vi "HFRR ADV v037.vi"() -> ()   [LabVIEW 2025] (continued)
                w348 = "" ("FILE")
                n261 = local write "Main Tab"(T2."Adv Scar" ("Main Tab")) -> ()
                n262 = local write "measured_stroke"(0.0 ("measured_stroke")) -> ()
                n263 = local write "Main Dashboard Buttons"(T1."Imaging" ("Main Dashboard Buttons")) -> ()
                n264 = property on="RUN" class="Bool (strict)"("Visible"=TRUE) -> ()  [unwired: 2 in, 2 out]
                n265 = local write "Due Write"("VC;0") -> ()
                n266 = local write "Humidity"(TRUE ("Humidity")) -> ()
                n267 = local write "TEST FILE NAM,E SAVED"(FALSE ("TEST FILE NAM,E SAVED")) -> ()
                n268 = local write "Fuel Discription :"(w348) -> ()
                n269 = local write "Batch Ref Num :"(w348) -> ()
                n270 = local write "Remarks :"(w348) -> ()
                n271 = local write "FILE"(w348) -> ()
                n272 = property on="FRICVALZ 2" class="Bool (strict)"("DisabledEnum"=w347) -> ()  [unwired: 2 in, 2 out]
                n273 = property on="FRICVALZ 4" class="Bool (strict)"("DisabledEnum"=w347) -> ()  [unwired: 2 in, 2 out]
                n274 = property on="FRICVALZ 3" class="Bool (strict)"("DisabledEnum"=w347) -> ()  [unwired: 2 in, 2 out]
              }
            }
          }
          frame True {
            n275 = stacked-sequence {
              frame #0 {
                n276 = local write "Due Write"("DAC;200") -> ()
              }
              frame #1 {
                n277 = Wait (ms)(milliseconds to wait=u32 1500) -> ()  [unwired: 1 out]
              }
              frame #2 {
                n278 = local write "Due Write"("DAC;200") -> ()
              }
              frame #3 {
                n279 = Wait (ms)(milliseconds to wait=u32 1000) -> ()  [unwired: 1 out]
              }
              frame #4 {
                n280 = local write "Due Write"("VC;1") -> ()
              }
              frame #5 {
                n281 = Wait (ms)(milliseconds to wait=u32 2000) -> ()  [unwired: 1 out]
              }
              frame #6 {
                n282 = local write "Due Write"("VC;1") -> ()
              }
              frame #7 {
                n283 = Wait (ms)(milliseconds to wait=u32 2000) -> ()  [unwired: 1 out]
              }
              frame #8 {
                w359 = T19."Disabled" ("Disabled")
                n284 = property on="RUN" class="Bool (strict)"("Visible"=FALSE) -> ()  [unwired: 2 in, 2 out]
                n285 = property on="FRICVALZ 2" class="Bool (strict)"("DisabledEnum"=w359) -> ()  [unwired: 2 in, 2 out]
                n286 = property on="FRICVALZ 4" class="Bool (strict)"("DisabledEnum"=w359) -> ()  [unwired: 2 in, 2 out]
                n287 = property on="FRICVALZ 3" class="Bool (strict)"("DisabledEnum"=w359) -> ()  [unwired: 2 in, 2 out]
                "START TEMP" <- TRUE
              }
            }
          }
        }
      }
      event "FILE", "USERNAME", "USER ID": Mouse Enter {
        n288 = event-data() -> ()  [unwired: 1 in, 4 out]
        n289 = dll-call lib="kernel32.dll" fn="Wow64DisableWow64FsRedirection"("OldValue"=0) -> (error out=w366:errorcluster, "OldValue"=w364:i32)  [unwired: 4 in, 1 out]
        n290 = call <vilib>:"System Exec.vi"("run minimized? (F)"=TRUE, "error in (no error)"=w366, "command line"="C:\\Program Files\\Common Files\\Microsoft Shared\\Ink\\TabTip.exe") -> ("error out"=w365:errorcluster)  [unwired: 5 in, 3 out]
        n291 = dll-call lib="kernel32.dll" fn="Wow64EnableWow64FsRedirection"(error in=w365, "OldValue"=w364) -> ()  [unwired: 4 in, 2 out]
      }
      event "EDIT": Value Change {
        n292 = event-data() -> ()  [unwired: 1 in, 6 out]
        n293 = local read "EDIT"() -> (w367:bool)
        n294 = case shown="False" w367 {
          frame False {
            n295 = control-ref of="This VI"() -> (w384:refnum<vi>)
            n296 = property class="VI"(reference=w384) -> (reference out=w375:refnum<vi>, error out=w379:errorcluster, "Panel"=w383:refnum<vi>)  [unwired: 1 in]
            n297 = property class="Pnl"(reference=w383, error in=w379) -> (reference out=w377:refnum<vi>, error out=w380:errorcluster, "Panes[]"=w382:refnum<vi>[])
            n298 = for {
              tunnel: w382 -> [w390] mode=indexing
              tunnel: T24."Always Off" ("Horizontal Scrollbar Visibility") -> [w389]
              tunnel: w380 -> [w386]
              tunnel: [w385] -> w378
              n299 = property class="Pane"(reference=w390, error in=w386, "HorizScrollbarVisibility"=w389) -> (reference out=w387:refnum<vi>, error out=w388:errorcluster)
              n300 = Close Reference(reference=w387, error in (no error)=w388) -> (error out=w385:errorcluster)
            }
            n301 = Close Reference(reference=w377, error in (no error)=w378) -> (error out=w376:errorcluster)
            n302 = Close Reference(reference=w375, error in (no error)=w376) -> (error out=w370:errorcluster)
            "error out 7" <- w370
            n303 = call <vilib>:"Clear Errors.vi"("error in (no error)"=w370) -> ("error out"=w369:errorcluster)  [unwired: 5 in, 1 out]
            n304 = local write "Service Password enable"(FALSE ("Service Password enable")) -> ()
            n305 = call <userlib>:"Fit VI window to Largest Dec.vi"("error in (no error)"=w369, "border spacing (2 px)"=1) -> ("error out"=w374:errorcluster, "dup VI Ref"=w372:refnum<vi>)  [unwired: 4 in]
            n306 = invoke on="Invoke Node" class="VI" method="FP.Run-Time Position.Maximized"(reference=w372, error in=w374) -> (error out=w373:errorcluster)  [unwired: 2 in, 3 out]
            n307 = call <vilib>:"Clear Errors.vi"("error in (no error)"=w373) -> ()  [unwired: 5 in, 2 out]
          }
          frame True {
          }
        }
      }
      event "Heater Button": Value Change {
        n308 = event-data() -> ()  [unwired: 1 in, 6 out]
        n309 = local read "Heater Button"() -> (w391:bool)
        n310 = case shown="True" w391 {
          frame True {
            n311 = stacked-sequence {
              frame #0 {
                n312 = Wait (ms)(milliseconds to wait=u32 1500) -> ()  [unwired: 1 out]
              }
              frame #1 {
                n313 = local read "Set Temp"() -> (w393:dbl)
                n314 = Number To Fractional String(number=w393, precision (6)=i16 2) -> (F-format string=w396:string)  [unwired: 2 in]
                n315 = Concatenate Strings("ST;" ("Command"), w396) -> (w395:string)
                n316 = local write "Due Write"(w395) -> ()
              }
              frame #2 {
                n317 = Wait (ms)(milliseconds to wait=u32 1500) -> ()  [unwired: 1 out]
              }
              frame #3 {
                n318 = local write "Due Write"("HE;1" ("Command")) -> ()
              }
              frame #4 {
                n319 = Wait (ms)(milliseconds to wait=u32 1500) -> ()  [unwired: 1 out]
              }
              frame #5 {
                n320 = stacked-sequence {
                  frame #0 {
                    n321 = Wait (ms)(milliseconds to wait=u32 1500) -> ()  [unwired: 1 out]
                  }
                  frame #1 {
                    n322 = local read "Set Temp"() -> (w402:dbl)
                    n323 = Number To Fractional String(number=w402, precision (6)=i16 2) -> (F-format string=w405:string)  [unwired: 2 in]
                    n324 = Concatenate Strings("ST;" ("Command"), w405) -> (w404:string)
                    n325 = local write "Due Write"(w404) -> ()
                  }
                  frame #2 {
                    n326 = Wait (ms)(milliseconds to wait=u32 1500) -> ()  [unwired: 1 out]
                  }
                  frame #3 {
                    n327 = local write "Due Write"("HE;1" ("Command")) -> ()
                  }
                  frame #4 {
                    n328 = Wait (ms)(milliseconds to wait=u32 1500) -> ()  [unwired: 1 out]
                  }
                }
              }
            }
          }
          frame False {
            n329 = stacked-sequence {
              frame #0 {
                n330 = Wait (ms)(milliseconds to wait=u32 1500) -> ()  [unwired: 1 out]
              }
              frame #1 {
                n331 = Concatenate Strings("ST;" ("Command"), "0" ("string")) -> (w412:string)
                n332 = local write "Due Write"(w412) -> ()
              }
              frame #2 {
                n333 = Wait (ms)(milliseconds to wait=u32 1500) -> ()  [unwired: 1 out]
              }
              frame #3 {
                n334 = local write "Due Write"("HE;0" ("Command")) -> ()
              }
              frame #4 {
                n335 = Wait (ms)(milliseconds to wait=u32 1500) -> ()  [unwired: 1 out]
              }
            }
          }
        }
      }
      event "Headen Service Button": Value Change {
        n336 = event-data() -> ()  [unwired: 1 in, 6 out]
        n337 = local read "Headen Service Button"() -> (w417:bool)
        n338 = case shown="True" w417 {
          frame False {
            n339 = property on="Password 3" class="Clust (strict)"("Visible"=FALSE) -> ()  [unwired: 2 in, 2 out]
            n340 = property on="Service Password Log" class="Str"("Visible"=FALSE) -> ()  [unwired: 2 in, 2 out]
          }
          frame True {
            n341 = property on="Password 3" class="Clust (strict)"("Visible"=TRUE) -> ()  [unwired: 2 in, 2 out]
            n342 = property on="Service Password Log" class="Str"("Visible"=TRUE) -> ()  [unwired: 2 in, 2 out]
          }
        }
      }
      event "Password 3.Service Password": Value Change {
        n343 = event-data() -> ()  [unwired: 1 in, 6 out]
        n344 = Unbundle By Name("Password 3") -> ("Service Password"=w424:string)
        n345 = call <vilib>:"Trim Whitespace.vi"("string"=w424) -> ("trimmed string"=w422:string)  [unwired: 1 in]
        n346 = Equal?(x=w422, y="Service@123") -> (x = y?=w423:bool)
        n347 = case shown="False" w423 {
          selector: w423 -> [w427 w429]
          frame False {
            n348 = local write "Service Password enable"(w427) -> ()
            n349 = property on="Service Password Log" class="Str"("Visible"=TRUE) -> ()  [unwired: 2 in, 2 out]
          }
          frame True {
            n350 = property on="Service Password Log" class="Str"("Visible"=FALSE) -> ()  [unwired: 2 in, 2 out]
            "Service Password enable" <- w429
          }
        }
      }
      event "Sign In": Value Change {
        w431 = FALSE ("Visible")
        n351 = event-data() -> ()  [unwired: 1 in, 6 out]
        n352 = property on="About" class="Clust (strict)"("Visible"=w431) -> ()  [unwired: 2 in, 2 out]
        n353 = property on="Password 3" class="Clust (strict)"("Visible"=w431) -> ()  [unwired: 2 in, 2 out]
        n354 = property on="Service Password Log" class="Str"("Visible"=FALSE) -> ()  [unwired: 2 in, 2 out]
      }
      event "Info": Value Change {
        n355 = event-data() -> ()  [unwired: 1 in, 6 out]
        n356 = local read "Info"() -> (w433:bool)
        n357 = case shown="False" w433 {
          frame False {
            n358 = property on="About" class="Clust (strict)"("Visible"=FALSE) -> ()  [unwired: 2 in, 2 out]
          }
          frame True {
            n359 = property on="About" class="Clust (strict)"("Visible"=TRUE) -> ()  [unwired: 2 in, 2 out]
          }
        }
      }
      event "Calibration": Value Change {
        n360 = event-data() -> ()  [unwired: 1 in, 6 out]
        n361 = local read "Calibration"() -> (w437:bool)
        n362 = case shown="False" w437 {
          frame False {
            n363 = property on="Calibration 2" class="TabCtl (strict)"("Visible"=FALSE) -> ()  [unwired: 2 in, 2 out]
            n364 = local write "Cal Password"("" ("Cal Password")) -> ()
          }
          frame True {
            n365 = property on="Calibration 2" class="TabCtl (strict)"("Visible"=TRUE) -> ()  [unwired: 2 in, 2 out]
            n366 = local write "Cal Password"("" ("Cal Password")) -> ()
          }
        }
        n367 = property on="Wrong Password" class="Str"("Visible"=FALSE) -> ()  [unwired: 2 in, 2 out]
      }
      event "Cal Password": Value Change {
        n368 = event-data() -> ()  [unwired: 1 in, 6 out]
        n369 = local read "Cal Password"() -> (w445:string)
        n370 = call <vilib>:"Trim Whitespace.vi"("string"=w445) -> ("trimmed string"=w444:string)  [unwired: 1 in]
        n371 = Equal?(x=w444, y="Cal@321") -> (x = y?=w442:bool)
        n372 = case shown="True" w442 {
          frame False {
            n373 = property on="Wrong Password" class="Str"("Visible"=TRUE) -> ()  [unwired: 2 in, 2 out]
          }
          frame True {
            n374 = property on="Wrong Password" class="Str"("Visible"=FALSE) -> ()  [unwired: 2 in, 2 out]
            n375 = local write "Main Tab"(T2."About" ("Main Tab")) -> ()
            n376 = local write "Cal Password"("" ("Cal Password")) -> ()
            n377 = local write "Main Dashboard Buttons"(T1."About" ("Main Dashboard Buttons")) -> ()
            n378 = property on="Calibration 2" class="TabCtl (strict)"("Visible"=FALSE) -> ()  [unwired: 2 in, 2 out]
            n379 = local write "Calibration"(FALSE ("Calibration")) -> ()
          }
        }
      }
      event "Calibration Selection": Value Change {
        n380 = event-data() -> ()  [unwired: 1 in, 6 out]
        n381 = local read "Calibration Selection"() -> (w454:T8)
        n382 = case shown="\"Stroke Calibration\"" w454 {
          tunnel: [T7."Stroke" ("Main Calibration Tab") T7."Friction" ("Main Calibration Tab") T7."Main" ("Main Calibration Tab") T7."Temperature" ("Main Calibration Tab")] -> w453
          frame "Stroke Calibration" {
          }
          frame "Friction Force Calibration" {
          }
          frame Default {
          }
          frame "Temperature Calibration" {
          }
        }
        n383 = local write "Main Calibration Tab"(w453) -> ()
      }
      event "Back Stroke": Value Change {
        n384 = event-data() -> ()  [unwired: 1 in, 6 out]
        n385 = local write "Main Stroke Tab"(T9."Step 1" ("Main Stroke Tab")) -> ()
        n386 = local write "Main Calibration Tab"(T7."Main" ("Main Calibration Tab")) -> ()
        n387 = local write "Back Stroke"(FALSE ("Back Stroke")) -> ()
      }
      event "Step 2 Back": Value Change {
        n388 = event-data() -> ()  [unwired: 1 in, 6 out]
        n389 = local write "Main Stroke Tab"(T9."Step 1" ("Main Stroke Tab")) -> ()
        n390 = local write "Step 2 Back"(FALSE ("Back Stroke")) -> ()
      }
      event "Step 3 Back": Value Change {
        n391 = event-data() -> ()  [unwired: 1 in, 6 out]
        n392 = local write "Main Stroke Tab"(T9."Step 2" ("Main Stroke Tab")) -> ()
        n393 = local write "Step 3 Back"(FALSE ("Back Stroke")) -> ()
      }
      event "Step 4 Back": Value Change {
        n394 = event-data() -> ()  [unwired: 1 in, 6 out]
        n395 = local write "Main Stroke Tab"(T9."Step 3" ("Main Stroke Tab")) -> ()
        n396 = local write "Step 4 Back"(FALSE ("Back Stroke")) -> ()
      }
      event "Step 5 Back": Value Change {
        n397 = event-data() -> ()  [unwired: 1 in, 6 out]
        n398 = local write "Main Stroke Tab"(T9."Step 4" ("Main Stroke Tab")) -> ()
        n399 = local write "Step 5 Back"(FALSE ("Back Stroke")) -> ()
      }
      event "Step 6 Back": Value Change {
        n400 = event-data() -> ()  [unwired: 1 in, 6 out]
        n401 = local write "Main Stroke Tab"(T9."Step 5" ("Main Stroke Tab")) -> ()
        n402 = local write "Step 6 Back"(FALSE ("Back Stroke")) -> ()
      }
      event "Back Stroke step 7": Value Change {
        n403 = event-data() -> ()  [unwired: 1 in, 6 out]
        n404 = local write "Main Stroke Tab"(T9."Step 6" ("Main Stroke Tab")) -> ()
        n405 = local write "Back Stroke step 7"(FALSE ("Back Stroke")) -> ()
      }
      event "Back Stroke step 8": Value Change {
        n406 = event-data() -> ()  [unwired: 1 in, 6 out]
        n407 = local write "Main Stroke Tab"(T9."Step 7" ("Main Stroke Tab")) -> ()
        n408 = local write "Back Stroke step 8"(FALSE ("Back Stroke")) -> ()
      }
      event "Back Stroke 8": Value Change {
        n409 = event-data() -> ()  [unwired: 1 in, 6 out]
        n410 = local write "MOVE CARRIAGE TO"(0.2 ("MOVE CARRIAGE TO")) -> ()
        n411 = local write "Main Stroke Tab"(T9."Step 1" ("Main Stroke Tab")) -> ()
        n412 = local write "Back Stroke 8"(FALSE ("Back Stroke 8")) -> ()
      }
      event "Continue Stroke": Value Change {
        n413 = event-data() -> ()  [unwired: 1 in, 6 out]
        n414 = local write "Main Stroke Tab"(T9."Step 2" ("Main Stroke Tab")) -> ()
        n415 = local write "Continue Stroke"(FALSE ("Continue Stroke")) -> ()
      }
      event "Continue Stroke step 2": Value Change {
        n416 = event-data() -> ()  [unwired: 1 in, 6 out]
        n417 = local write "Main Stroke Tab"(T9."Step 3" ("Main Stroke Tab")) -> ()
        n418 = local write "Continue Stroke step 2"(FALSE ("Continue Stroke")) -> ()
      }
      event "Continue Stroke step 3": Value Change {
        n419 = event-data() -> ()  [unwired: 1 in, 6 out]
        n420 = local write "Main Stroke Tab"(T9."Step 4" ("Main Stroke Tab")) -> ()
        n421 = local write "Continue Stroke step 3"(FALSE ("Continue Stroke")) -> ()
      }
      event "Continue Stroke step 4": Value Change {
        n422 = event-data() -> ()  [unwired: 1 in, 6 out]
        n423 = local write "Main Stroke Tab"(T9."Step 5" ("Main Stroke Tab")) -> ()
        n424 = local write "Continue Stroke step 4"(FALSE ("Continue Stroke")) -> ()
      }
      event "Continue Stroke step 5": Value Change {
        n425 = event-data() -> ()  [unwired: 1 in, 6 out]
        n426 = local write "Main Stroke Tab"(T9."Step 6" ("Main Stroke Tab")) -> ()
        n427 = local write "Continue Stroke step 5"(FALSE ("Continue Stroke")) -> ()
      }
      event "Continue Stroke step 6": Value Change {
        n428 = event-data() -> ()  [unwired: 1 in, 6 out]
        n429 = local write "Main Stroke Tab"(T9."Step 7" ("Main Stroke Tab")) -> ()
        n430 = local write "Continue Stroke step 6"(FALSE ("Continue Stroke")) -> ()
      }
      event "Continue Stroke step 7": Value Change {
        w493 = FALSE ("0.2mm")
        n431 = event-data() -> ()  [unwired: 1 in, 6 out]
        n432 = local write "0.4 mm"(w493) -> ()
        n433 = local write "0.6 mm"(w493) -> ()
        n434 = local write "1.0 mm"(w493) -> ()
        n435 = local write "1.2 mm"(w493) -> ()
        n436 = local write "0.2 2"(w493) -> ()
        n437 = local write "0.4 2"(w493) -> ()
        n438 = local write "0.6 2"(w493) -> ()
        n439 = local write "0.8 2"(w493) -> ()
        n440 = local write "1.0 2"(w493) -> ()
        n441 = local write "1.2"(w493) -> ()
        n442 = local write "0.2mm"(w493) -> ()
        n443 = local write "0.8mm"(w493) -> ()
        n444 = local write "Main Stroke Tab"(T9."Step 8" ("Main Stroke Tab")) -> ()
        n445 = local write "Continue Stroke step 7"(FALSE ("Continue Stroke")) -> ()
        n446 = local write "Stroke Test Complete"(T10."Test Progress" ("Stroke Test Complete")) -> ()
        "Position Measurment Temp" <- 0.0 ("Position Measurment Temp")
        "Calibration Tare" <- TRUE ("Calibration Tare")
        "MOVE CARRIAGE TO" <- 0.2 ("MOVE CARRIAGE TO")
      }
      event "Continue Stroke step 8": Value Change {
        n447 = event-data() -> ()  [unwired: 1 in, 6 out]
        n448 = local read "LVDT STROKE  Calibration"() -> (w498:dbl)
        n449 = local read "Position Measurment Temp"() -> (w499:dbl)
        n450 = case shown="7" w499 {
          selector: w499 -> [w504 w509 w514 w519 w524 w528 w531 w532]
          tunnel: w498 -> [w500 w505 w510 w515 w520 w525 _ _]
          frame 0, Default {
            w502 = TRUE ("0.2mm")
            n451 = Increment(x=w504) -> (x+1=w503:i32)
            n452 = local write "Position Measurment Temp"(w503) -> ()
            n453 = local write "0.2mm"(w502) -> ()
            n454 = local write "0.2 2"(w502) -> ()
            n455 = local write "MOVE CARRIAGE TO"(0.4 ("MOVE CARRIAGE TO")) -> ()
            "Calibration 0.2" <- w500
          }
          frame 1 {
            w507 = TRUE ("0.4 mm")
            n456 = Increment(x=w509) -> (x+1=w508:i32)
            n457 = local write "Calibration 0.4"(w505) -> ()
            n458 = local write "Position Measurment Temp"(w508) -> ()
            n459 = local write "0.4 mm"(w507) -> ()
            n460 = local write "MOVE CARRIAGE TO"(0.6 ("MOVE CARRIAGE TO")) -> ()
            n461 = local write "0.4 2"(w507) -> ()
          }
          frame 2 {
            w512 = TRUE ("0.6 mm")
            n462 = Increment(x=w514) -> (x+1=w513:i32)
            n463 = local write "Calibration 0.6"(w510) -> ()
            n464 = local write "Position Measurment Temp"(w513) -> ()
            n465 = local write "0.6 2"(w512) -> ()
            n466 = local write "0.6 mm"(w512) -> ()
            n467 = local write "MOVE CARRIAGE TO"(0.8 ("MOVE CARRIAGE TO")) -> ()
          }
          frame 3 {
            w516 = TRUE ("0.6 mm")
            n468 = Increment(x=w519) -> (x+1=w518:i32)
            n469 = local write "Position Measurment Temp"(w518) -> ()
            n470 = local write "MOVE CARRIAGE TO"(1.0 ("MOVE CARRIAGE TO")) -> ()
            n471 = local write "0.8mm"(w516) -> ()
            n472 = local write "0.8 2"(w516) -> ()
            "Calibration 0.8" <- w515
          }
          frame 4 {
            w521 = TRUE ("0.6 mm")
            n473 = Increment(x=w524) -> (x+1=w523:i32)
            n474 = local write "Position Measurment Temp"(w523) -> ()
            n475 = local write "MOVE CARRIAGE TO"(1.2 ("MOVE CARRIAGE TO")) -> ()
            n476 = local write "1.0 mm"(w521) -> ()
            n477 = local write "1.0 2"(w521) -> ()
            "Calibration 1.0" <- w520
          }
          frame 5 {
            w526 = TRUE ("0.6 mm")
            n478 = Increment(x=w528) -> (x+1=w527:i32)
            n479 = local write "Position Measurment Temp"(w527) -> ()
            n480 = local write "1.2 mm"(w526) -> ()
            n481 = local write "1.2"(w526) -> ()
            "Calibration 1.2" <- w525
          }
          frame 6 {
            n482 = Increment(x=w531) -> (x+1=w530:i32)
            n483 = local write "Position Measurment Temp"(w530) -> ()
            n484 = local write "Stroke Test Complete"(T10."Stroke Points Completed" ("Stroke Test Complete")) -> ()
          }
          frame 7 {
            n485 = stacked-sequence {
              tunnel: w532 -> [w533 _ _]
              frame #0 {
                n486 = Increment(x=w533) -> (x+1=w534:i32)
                n487 = local write "Main Stroke Tab"(T9."Step 9" ("Main Stroke Tab")) -> ()
                n488 = local write "Position Measurment Temp"(w534) -> ()
                n489 = Insert Into Array(array=dbl[] [], new element #1=0.2 ("new element/subarray"), new element #2=0.4 ("new element/subarray"), new element #3=0.6 ("new element/subarray"), new element #4=0.8 ("new element/subarray"), new element #5=1.0 ("new element/subarray"), new element #6=1.2 ("new element/subarray")) -> (→"1D stroke":dbl[])  [unwired: 1 in]
                n490 = local read "Calibration 0.2"() -> (w541:dbl)
                n491 = local read "Calibration 0.4"() -> (w540:dbl)
                n492 = local read "Calibration 0.6"() -> (w539:dbl)
                n493 = local read "Calibration 0.8"() -> (w538:dbl)
                n494 = local read "Calibration 1.0"() -> (w537:dbl)
                n495 = local read "Calibration 1.2"() -> (w536:dbl)
                n496 = Insert Into Array(array=dbl[] [], new element #1=w541, new element #2=w540, new element #3=w539, new element #4=w538, new element #5=w537, new element #6=w536) -> (→"Calibrated Voltage Value":dbl[])  [unwired: 1 in]
              }
              frame #1 {
                n497 = local read "calibration values"() -> (w564:dbl[])
                n498 = local read "Calibrated Voltage Value"() -> (w566:dbl[])
                n499 = Index Array(array=w564, index #1=1 ("index"), index #2=3 ("index"), index #3=5 ("index"), index #4=7 ("index"), index #5=9 ("index"), index #6=11 ("index")) -> (element #1=w557:dbl, element #2=w556:dbl, element #3=w555:dbl, element #4=w554:dbl, element #5=w553:dbl, element #6=w552:dbl)
                n500 = local read "1D stroke"() -> (w567:dbl[])
                n501 = for {
                  tunnel: [w576] -> w565 mode=indexing
                  tunnel: w567 -> [w575] mode=indexing
                  tunnel: w566 -> [w574] mode=indexing
                  tunnel: w557 -> [w573]
                  tunnel: w556 -> [w572]
                  tunnel: w555 -> [w571]
                  tunnel: w554 -> [w570]
                  tunnel: w553 -> [w569]
                  tunnel: w552 -> [w568]
                  n502 = formula code="if (stroke == 0.2)\n{\n    if ((voltage >= REF_02 - 0.2) && (voltage <= REF_02 + 0.2))\n        status = 1;\n    else\n        status = 0;\n}\nelse if (stroke == 0.4)\n{\n    if ((voltage >= REF_04 - 0.2) && (voltage <= REF_04 + 0.2))\n        status = 1;\n    else\n        status = 0;\n}\nelse if (stroke == 0.6)\n{\n    if ((voltage >= REF_06 - 0.2) && (voltage <= REF_06 + 0.2))\n        status = 1;\n    else\n        status = 0;\n}\nelse if (stroke == 0.8)\n{\n    if ((voltage >= REF_08 - 0.2) && (voltage <= REF_08 + 0.2))\n        status = 1;\n    else\n        status = 0;\n}\nelse if (stroke == 1.0)\n{\n    if ((voltage >= REF_10 - 0.2) && (voltage <= REF_10 + 0.2))\n        status = 1;\n    else\n        status = 0;\n}\nelse if (stroke == 1.2)\n{\n    if ((voltage >= REF_12 - 0.2) && (voltage <= REF_12 + 0.2))\n        status = 1;\n    else\n        status = 0;\n}\nelse\n{\n    status = 0;\n}"("stroke"=w575, "voltage"=w574, "REF_02"=w573, "REF_04"=w572, "REF_06"=w571, "REF_08"=w570, "REF_10"=w569, "REF_12"=w568) -> ("status"=w576:dbl)
                }
                "Status" <- w565
              }
              frame #2 {
                w583 = 1.0
                n503 = local read "Status"() -> (w590:dbl[])
                n504 = Index Array(array=w590) -> (element #1=w589:dbl, element #2=w588:dbl, element #3=w587:dbl, element #4=w586:dbl, element #5=w585:dbl, element #6=w584:dbl)  [unwired: 6 in]
                n505 = Equal?(x=w588, y=w583) -> (x = y?=w581:bool)
                n506 = Equal?(x=w587, y=w583) -> (x = y?=w580:bool)
                n507 = Equal?(x=w586, y=w583) -> (x = y?=w579:bool)
                n508 = Equal?(x=w585, y=w583) -> (x = y?=w578:bool)
                n509 = Equal?(x=w584, y=w583) -> (x = y?=w577:bool)
                n510 = Equal?(x=w589, y=w583) -> (x = y?=w582:bool)
                n511 = case shown="True" w582 {
                  selector: w582 -> [w601 w602]
                  frame True {
                    n512 = local write "Point 1 - 0.2 mm"(w601) -> ()
                    n513 = property on="Point 1 - 0.2 mm" class="Bool"("Caption.Visible"=w601) -> ()  [unwired: 2 in, 2 out]
                  }
                  frame False {
                    n514 = local write "Point 1 - 0.2 mm"(w602) -> ()
                    n515 = property on="Point 1 - 0.2 mm" class="Bool"("Caption.Visible"=w602) -> ()  [unwired: 2 in, 2 out]
                  }
                }
                n516 = case shown="True" w581 {
                  selector: w581 -> [w599 w600]
                  frame True {
                    n517 = local write "Point 2 - 0.4 mm"(w599) -> ()
                    n518 = property on="Point 2 - 0.4 mm" class="Bool"("Caption.Visible"=w599) -> ()  [unwired: 2 in, 2 out]
                  }
                  frame False {
                    n519 = local write "Point 2 - 0.4 mm"(w600) -> ()
                    n520 = property on="Point 2 - 0.4 mm" class="Bool"("Caption.Visible"=w600) -> ()  [unwired: 2 in, 2 out]
                  }
                }
                n521 = case shown="True" w578 {
                  selector: w578 -> [w593 w594]
                  frame True {
                    n522 = local write "Point 5 - 1.0 mm"(w593) -> ()
                    n523 = property on="Point 5 - 1.0 mm" class="Bool"("Caption.Visible"=w593) -> ()  [unwired: 2 in, 2 out]
                  }
                  frame False {
                    n524 = local write "Point 5 - 1.0 mm"(w594) -> ()
                    n525 = property on="Point 5 - 1.0 mm" class="Bool"("Caption.Visible"=w594) -> ()  [unwired: 2 in, 2 out]
                  }
                }
                n526 = case shown="True" w580 {
                  selector: w580 -> [w597 w598]
                  frame True {
                    n527 = local write "Point 3 - 0.6 mm"(w597) -> ()
                    n528 = property on="Point 3 - 0.6 mm" class="Bool"("Caption.Visible"=w597) -> ()  [unwired: 2 in, 2 out]
                  }
                  frame False {
                    n529 = local write "Point 3 - 0.6 mm"(w598) -> ()
                    n530 = property on="Point 3 - 0.6 mm" class="Bool"("Caption.Visible"=w598) -> ()  [unwired: 2 in, 2 out]
                  }
                }
                n531 = case shown="True" w579 {
                  selector: w579 -> [w595 w596]
                  frame True {
                    n532 = local write "Point 4 - 0.8 mm"(w595) -> ()
                    n533 = property on="Point 4 - 0.8 mm" class="Bool"("Caption.Visible"=w595) -> ()  [unwired: 2 in, 2 out]
                  }
                  frame False {
                    n534 = local write "Point 4 - 0.8 mm"(w596) -> ()
                    n535 = property on="Point 4 - 0.8 mm" class="Bool"("Caption.Visible"=w596) -> ()  [unwired: 2 in, 2 out]
                  }
                }
                n536 = case shown="True" w577 {
                  selector: w577 -> [w591 w592]
                  frame True {
                    n537 = local write "Point 6 - 1.2 mm"(w591) -> ()
                    n538 = property on="Point 6 - 1.2 mm" class="Bool"("Caption.Visible"=w591) -> ()  [unwired: 2 in, 2 out]
                  }
                  frame False {
                    n539 = local write "Point 6 - 1.2 mm"(w592) -> ()
                    n540 = property on="Point 6 - 1.2 mm" class="Bool"("Caption.Visible"=w592) -> ()  [unwired: 2 in, 2 out]
                  }
                }
              }
            }
          }
        }
      }
      event "TEMPERATURE STEP Back 1", "TEMPERATURE STEP Back air Temp": Value Change {
        n541 = event-data() -> ()  [unwired: 1 in, 6 out]
        n542 = stacked-sequence {
          frame #0 {
            n543 = local write "Main Calibration Tab"(T7."Main" ("Main Calibration Tab")) -> ()
          }
          frame #1 {
            n544 = Wait (ms)(milliseconds to wait=u32 1000) -> ()  [unwired: 1 out]
          }
          frame #2 {
            n545 = local write "Due Write"("CAL;END" ("Command")) -> ()
          }
          frame #3 {
            n546 = Wait (ms)(milliseconds to wait=u32 2000) -> ()  [unwired: 1 out]
          }
          frame #4 {
            n547 = local write "Due Write"("CAL;END" ("Command")) -> ()
          }
        }
      }
      event "Temperature Continue Step 1": Value Change {
        n548 = event-data() -> ()  [unwired: 1 in, 6 out]
        n549 = stacked-sequence {
          frame #0 {
            n550 = Wait (ms)(milliseconds to wait=u32 1500) -> ()  [unwired: 1 out]
          }
          frame #1 {
            n551 = local write "Due Write"("CAL;START" ("Command")) -> ()
          }
          frame #2 {
            n552 = Wait (ms)(milliseconds to wait=u32 1500) -> ()  [unwired: 1 out]
          }
          frame #3 {
            n553 = local write "Due Write"("CAL;START" ("Command")) -> ()
          }
          frame #4 {
            n554 = Wait (ms)(milliseconds to wait=u32 2000) -> ()  [unwired: 1 out]
          }
          frame #5 {
          }
          frame #6 {
            n555 = Wait (ms)(milliseconds to wait=u32 2000) -> ()  [unwired: 1 out]
          }
          frame #7 {
            # "CAL;A1;<true_T>"
            n556 = local write "Due Write"("CAL;A1;0" ("Command")) -> ()
          }
          frame #8 {
            n557 = local write "Tab Control 4"(T12."Step 2" ("Tab Control 4")) -> ()
          }
        }
      }
      event "Temperature Continue Step air Step 1": Value Change {
        n558 = event-data() -> ()  [unwired: 1 in, 6 out]
        n559 = stacked-sequence {
          frame #0 {
            n560 = Wait (ms)(milliseconds to wait=u32 1500) -> ()  [unwired: 1 out]
          }
          frame #1 {
            n561 = local write "Due Write"("CAL;START" ("Command")) -> ()
          }
          frame #2 {
            n562 = Wait (ms)(milliseconds to wait=u32 1500) -> ()  [unwired: 1 out]
          }
          frame #3 {
            n563 = local write "Due Write"("CAL;START" ("Command")) -> ()
          }
          frame #4 {
            n564 = Wait (ms)(milliseconds to wait=u32 2000) -> ()  [unwired: 1 out]
          }
          frame #5 {
          }
          frame #6 {
            n565 = Wait (ms)(milliseconds to wait=u32 2000) -> ()  [unwired: 1 out]
          }
          frame #7 {
            # "CAL;A1;<true_T>"
            n566 = local write "Due Write"("CAL;A1;0" ("Command")) -> ()
          }
          frame #8 {
            n567 = local write "Tab Control 4"(T12."Air Step 2" ("Tab Control 4")) -> ()
          }
        }
      }
      event "Temperature Selection": Value Change {
        n568 = event-data() -> ()  [unwired: 1 in, 6 out]
        n569 = local read "Temperature Selection"() -> (w624:T13)
        n570 = case shown="\"Sample Temperature\"" w624 {
          frame "Air Temperature" {
            n571 = local write "Tab Control 4"(T12."Air Step 1" ("Tab Control 4")) -> ()
          }
          frame "Sample Temperature" {
            n572 = local write "Tab Control 4"(T12."Step 1" ("Tab Control 4")) -> ()
          }
          frame "Default", Default {
          }
        }
      }
      event "Temperature Continue Step 2": Value Change {
        n573 = event-data() -> ()  [unwired: 1 in, 6 out]
        n574 = stacked-sequence {
          frame #0 {
            n575 = stacked-sequence {
              frame #0 {
                n576 = Wait (ms)(milliseconds to wait=u32 1500) -> ()  [unwired: 1 out]
              }
              frame #1 {
                # "CAL;A1;<true_T>"
                n577 = local write "Due Write"("CAL;A1;0" ("Command")) -> ()
              }
              frame #2 {
                n578 = Wait (ms)(milliseconds to wait=u32 1500) -> ()  [unwired: 1 out]
              }
              frame #3 {
                # "CAL;A1;<true_T>"
                n579 = local write "Due Write"("CAL;A1;0" ("Command")) -> ()
              }
              frame #4 {
              }
            }
          }
          frame #1 {
            n580 = local write "Tab Control 4"(T12."Step 3" ("Tab Control 4")) -> ()
          }
        }
      }
      event "Temperature Continue Step 5": Value Change {
        n581 = event-data() -> ()  [unwired: 1 in, 6 out]
        n582 = stacked-sequence {
          frame #0 {
            n583 = stacked-sequence {
              frame #0 {
                n584 = Wait (ms)(milliseconds to wait=u32 1500) -> ()  [unwired: 1 out]
              }
              frame #1 {
                # "CAL;A1;<true_T>"
                n585 = local write "Due Write"("CAL;A1;0" ("Command")) -> ()
              }
              frame #2 {
                n586 = Wait (ms)(milliseconds to wait=u32 1500) -> ()  [unwired: 1 out]
              }
              frame #3 {
                # "CAL;A1;<true_T>"
                n587 = local write "Due Write"("CAL;A1;0" ("Command")) -> ()
              }
              frame #4 {
              }
            }
          }
          frame #1 {
            n588 = local write "Tab Control 4"(T12."Air Step 3" ("Tab Control 4")) -> ()
          }
        }
      }
      event "Temperature Continue Step 3": Value Change {
        n589 = event-data() -> ()  [unwired: 1 in, 6 out]
        n590 = stacked-sequence {
          frame #0 {
            n591 = stacked-sequence {
              frame #0 {
                n592 = Wait (ms)(milliseconds to wait=u32 1500) -> ()  [unwired: 1 out]
              }
              frame #1 {
              }
              frame #2 {
              }
              frame #3 {
                # "CAL;A1;<true_T>"
                n593 = local write "Due Write"("CAL;A1;60" ("Command")) -> ()
              }
              frame #4 {
                n594 = Wait (ms)(milliseconds to wait=u32 2000) -> ()  [unwired: 1 out]
              }
              frame #5 {
                # "CAL;A1;<true_T>"
                n595 = local write "Due Write"("CAL;A1;60" ("Command")) -> ()
              }
            }
          }
          frame #1 {
            n596 = Wait (ms)(milliseconds to wait=u32 1000) -> ()  [unwired: 1 out]
          }
          frame #2 {
            n597 = local write "Due Write"("CAL;SAVE" ("Command")) -> ()
          }
          frame #3 {
            n598 = Wait (ms)(milliseconds to wait=u32 1000) -> ()  [unwired: 1 out]
          }
          frame #4 {
            n599 = local write "Due Write"("CAL;SAVE" ("Command")) -> ()
          }
          frame #5 {
            n600 = Wait (ms)(milliseconds to wait=u32 1000) -> ()  [unwired: 1 out]
          }
          frame #6 {
            # "CAL;END"
            n601 = local write "Due Write"("CAL;END" ("Command")) -> ()
          }
          frame #7 {
            n602 = Wait (ms)(milliseconds to wait=u32 1000) -> ()  [unwired: 1 out]
          }
          frame #8 {
            # "CAL;END"
            n603 = local write "Due Write"("CAL;END" ("Command")) -> ()
          }
          frame #9 {
            n604 = local write "Main Calibration Tab"(T7."Temperature" ("Main Calibration Tab")) -> ()
            n605 = local write "Tab Control 4"(T12."Main" ("Tab Control 4")) -> ()
          }
        }
      }
      event "Temperature Continue Step 6": Value Change {
        n606 = event-data() -> ()  [unwired: 1 in, 6 out]
        n607 = stacked-sequence {
          frame #0 {
            n608 = stacked-sequence {
              frame #0 {
                n609 = Wait (ms)(milliseconds to wait=u32 1500) -> ()  [unwired: 1 out]
              }
              frame #1 {
              }
              frame #2 {
              }
              frame #3 {
                # "CAL;A1;<true_T>"
                n610 = local write "Due Write"("CAL;A1;60" ("Command")) -> ()
              }
              frame #4 {
                n611 = Wait (ms)(milliseconds to wait=u32 2000) -> ()  [unwired: 1 out]
              }
              frame #5 {
                # "CAL;A1;<true_T>"
                n612 = local write "Due Write"("CAL;A1;60" ("Command")) -> ()
              }
            }
          }
          frame #1 {
            n613 = Wait (ms)(milliseconds to wait=u32 1000) -> ()  [unwired: 1 out]
          }
          frame #2 {
            n614 = local write "Due Write"("CAL;SAVE" ("Command")) -> ()
          }
          frame #3 {
            n615 = Wait (ms)(milliseconds to wait=u32 1000) -> ()  [unwired: 1 out]
          }
          frame #4 {
            n616 = local write "Due Write"("CAL;SAVE" ("Command")) -> ()
          }
          frame #5 {
            n617 = Wait (ms)(milliseconds to wait=u32 1000) -> ()  [unwired: 1 out]
          }
          frame #6 {
            # "CAL;END"
            n618 = local write "Due Write"("CAL;END" ("Command")) -> ()
          }
          frame #7 {
            n619 = Wait (ms)(milliseconds to wait=u32 1000) -> ()  [unwired: 1 out]
          }
          frame #8 {
            # "CAL;END"
            n620 = local write "Due Write"("CAL;END" ("Command")) -> ()
          }
          frame #9 {
            n621 = local write "Main Calibration Tab"(T7."Temperature" ("Main Calibration Tab")) -> ()
            n622 = local write "Tab Control 4"(T12."Main" ("Tab Control 4")) -> ()
          }
        }
      }
      event "Back Stroke step main temperature": Value Change {
        n623 = event-data() -> ()  [unwired: 1 in, 6 out]
        n624 = stacked-sequence {
          frame #0 {
            n625 = Wait (ms)(milliseconds to wait=u32 1000) -> ()  [unwired: 1 out]
          }
          frame #1 {
            # "CAL;END"
            n626 = local write "Due Write"("CAL;END" ("Command")) -> ()
          }
          frame #2 {
            n627 = Wait (ms)(milliseconds to wait=u32 1000) -> ()  [unwired: 1 out]
          }
          frame #3 {
            # "CAL;END"
            n628 = local write "Due Write"("CAL;END" ("Command")) -> ()
          }
          frame #4 {
            n629 = local write "Main Calibration Tab"(T7."Main" ("Main Calibration Tab")) -> ()
            n630 = local write "Tab Control 4"(T12."Main" ("Tab Control 4")) -> ()
          }
        }
      }
      event "TEMPERATURE STEP  Back 4", "TEMPERATURE STEP 1 Back 3", "TEMPERATURE STEP  Back 3", "TEMPERATURE STEP 1 Back 2": Value Change {
        # "Back Stroke step main temperature"
        n631 = event-data() -> ()  [unwired: 1 in, 6 out]
        n632 = stacked-sequence {
          frame #0 {
            n633 = Wait (ms)(milliseconds to wait=u32 1000) -> ()  [unwired: 1 out]
          }
          frame #1 {
            # "CAL;END"
            n634 = local write "Due Write"("CAL;END" ("Command")) -> ()
          }
          frame #2 {
            n635 = Wait (ms)(milliseconds to wait=u32 1000) -> ()  [unwired: 1 out]
          }
          frame #3 {
            # "CAL;END"
            n636 = local write "Due Write"("CAL;END" ("Command")) -> ()
          }
          frame #4 {
            # "TEMPERATURE STEP  Back 4"
            n637 = local write "Main Calibration Tab"(T7."Temperature" ("Main Calibration Tab")) -> ()
            n638 = local write "Tab Control 4"(T12."Main" ("Tab Control 4")) -> ()
          }
        }
      }
      event "FF BACK", "FF BACK 2", "FF BACK 3", "FF BACK 4", "FF BACK 5", "FF BACK 6": Value Change {
        n639 = event-data() -> ()  [unwired: 1 in, 6 out]
        n640 = stacked-sequence {
          frame #0 {
            n641 = Wait (ms)(milliseconds to wait=u32 1500) -> ()  [unwired: 1 out]
          }
          frame #1 {
            n642 = local write "Due Write"("VC;0") -> ()
          }
          frame #2 {
            n643 = Wait (ms)(milliseconds to wait=u32 1500) -> ()  [unwired: 1 out]
          }
          frame #3 {
            n644 = local write "Due Write"("VC;0") -> ()
          }
          frame #4 {
            w681 = FALSE
            n645 = local write "FF BACK 2"(w681) -> ()
            n646 = local write "FF BACK 3"(w681) -> ()
            n647 = local write "FF BACK 4"(w681) -> ()
            n648 = local write "FF BACK 5"(w681) -> ()
            n649 = local write "FF BACK 6"(w681) -> ()
            n650 = local write "FF BACK"(w681) -> ()
          }
          frame #5 {
            n651 = local write "Friction Force Tab"(T25."Page 1" ("Friction Force Tab")) -> ()
            n652 = local write "Main Calibration Tab"(T7."Main" ("Main Calibration Tab")) -> ()
          }
        }
      }
      event "FF CONTINUE": Value Change {
        n653 = event-data() -> ()  [unwired: 1 in, 6 out]
        n654 = local write "FF CONTINUE"(FALSE ("FF CONTINUE")) -> ()
        n655 = local write "Friction Force Tab"(T25."Page 2" ("Friction Force Tab")) -> ()
      }
      event "FF CONTINUE 2": Value Change {
        n656 = event-data() -> ()  [unwired: 1 in, 6 out]
        n657 = local write "FF CONTINUE 2"(FALSE ("FF CONTINUE")) -> ()
        n658 = local write "Friction Force Tab"(T25."Page 3" ("Friction Force Tab")) -> ()
      }
      event "FF CONTINUE 3": Value Change {
        n659 = event-data() -> ()  [unwired: 1 in, 6 out]
        n660 = local write "FF CONTINUE 3"(FALSE ("FF CONTINUE")) -> ()
        n661 = local write "Friction Force Tab"(T25."Page 4" ("Friction Force Tab")) -> ()
      }
      event "FF CONTINUE 4": Value Change {
        n662 = event-data() -> ()  [unwired: 1 in, 6 out]
        n663 = local write "FF CONTINUE 4"(FALSE ("FF CONTINUE")) -> ()
        n664 = local write "Friction Force Tab"(T25."Page 5" ("Friction Force Tab")) -> ()
      }
      event "FF CONTINUE 5": Value Change {
        n665 = event-data() -> ()  [unwired: 1 in, 6 out]
        n666 = local write "FF CONTINUE 5"(FALSE ("FF CONTINUE")) -> ()
        n667 = local write "Friction Force Tab"(T25."Page 6" ("Friction Force Tab")) -> ()
      }
      event "Quit": Value Change {
        n668 = event-data() -> ()  [unwired: 1 in, 6 out]
      }
    }
    n669 = Wait (ms)(milliseconds to wait=u32 100) -> ()  [unwired: 1 out]
  }
  n670 = while {
    stop <- w714 stop-if-true
    n671 = local read "Ambient Temperature"() -> (w712:dbl)
    n672 = local read "Sample Temperature"() -> (w711:dbl)
    n673 = Wait (ms)(milliseconds to wait=u32 200) -> ()  [unwired: 1 out]
    n674 = local write "Temperature — Live (Set A: 0 °C)"(w712) -> ()
    n675 = local write "Temperature — Live (Set A: 60 °C)"(w712) -> ()
    n676 = local write "Sensor value"(w712) -> ()
    n677 = local write "Sensor value"(w712) -> ()
    n678 = local write "Sensor value"(w711) -> ()
    n679 = local write "Sensor value"(w711) -> ()
    n680 = local write "Temperature — Live (Set A: 60 °C)"(w711) -> ()
    n681 = local write "Temperature — Live (Set A: 0 °C)"(w711) -> ()
    n682 = case shown="True" "Save Button" {
      selector: "Save Button" -> [_ w729]
      frame False {
      }
      frame True {
        n683 = Not(x=w729) -> (.not. x?=w728:bool)
        n684 = local read "milliseconds to wait"() -> (w761:u32)
        n685 = local read "max_step_change"() -> (w766:dbl)
        n686 = local read "max_amplitude"() -> (w767:dbl)
        n687 = local read "min_amplitude"() -> (w768:dbl)
        n688 = local read "PIEZO_CAL_FACTOR"() -> (w772:dbl)
        n689 = local write "Save Button"(w728) -> ()
        n690 = local read "startup_cmd"() -> (w769:dbl)
        n691 = local read "NORMAL_FORCE"() -> (w773:dbl)
        n692 = local read "ADC_Resolution"() -> (w771:dbl)
        n693 = local read "calibration values"() -> (w776:dbl[])
        n694 = local read "kp"() -> (w763:dbl)
        n695 = local read "kd"() -> (w765:dbl)
        n696 = local read "dt"() -> (w762:dbl)
        n697 = local read "ki"() -> (w764:dbl)
        n698 = local read "STROKE FILTER"() -> (w774:i32)
        n699 = local read "Add up Stroke"() -> (w775:dbl)
        n700 = local read "VREF"() -> (w770:dbl)
        n701 = Insert Into Array(array=dbl[] [], new element #1=w761, new element #2=w762, new element #3=w763, new element #4=w764, new element #5=w765, new element #6=w766, new element #7=w767, new element #8=w768, new element #9=w769) -> (w777:dbl[])  [unwired: 1 in]
        n702 = Insert Into Array(array=dbl[] [], new element #1=w770, new element #2=w771, new element #3=w772, new element #4=w773) -> (w778:dbl[])  [unwired: 1 in]
        n703 = Array To Spreadsheet String(delimiter (Tab)=";", array=w776, 3:"" ("format string")) -> (spreadsheet string=w780:string)
        n704 = Insert Into Array(array=dbl[] [], new element #1=w774, new element #2=w775) -> (w779:dbl[])  [unwired: 1 in]
        n705 = call "Write Config.vi"("Stroke Calibration"=w780, "STROKE PARAMETERS"=w779, "ADC PARAMETERS"=w778, "PID  PARAMETERS"=w777) -> ("error out"=w759:errorcluster)  [unwired: 7 in]
        n706 = call "Stall Data Flow.vim"("value in"=w759, "milliseconds to wait"=u32 2000) -> ("value out"=w760:errorcluster)  [unwired: 1 out]
        n707 = call "Read Config.vi"("error in (no error)"=w760) -> ("STROKE PARAMETERS"=w757:dbl[], "ADC PARAMETERS"=w756:dbl[], "PID  PARAMETERS"=w755:dbl[], "Stroke Calibration"=w758:string)  [unwired: 6 in, 1 out]
        n708 = Index Array(array=w755) -> (element #1=w753:dbl, element #2=w752:dbl, element #3=w751:dbl, element #4=w750:dbl, element #5=w749:dbl, element #6=w748:dbl, element #7=w747:dbl, element #8=w746:dbl, element #9=w745:dbl)  [unwired: 9 in]
        n709 = Index Array(array=w756) -> (element #1=w744:dbl, element #2=w743:dbl, element #3=w742:dbl, element #4=w741:dbl)  [unwired: 4 in]
        n710 = Index Array(array=w757) -> (element #1=w740:dbl, element #2=w739:dbl)  [unwired: 2 in]
        n711 = Spreadsheet String To Array(delimiter (Tab)=";", format string="", spreadsheet string=w758, array type (2D Dbl)=dbl[] []) -> (array=w754:dbl[])
        n712 = local write "VREF"(w744) -> ()
        n713 = local write "ADC_Resolution"(w743) -> ()
        n714 = local write "PIEZO_CAL_FACTOR"(w742) -> ()
        n715 = local write "NORMAL_FORCE"(w741) -> ()
        n716 = local write "STROKE FILTER"(w740) -> ()
        n717 = local write "Add up Stroke"(w739) -> ()
        n718 = local write "calibration values"(w754) -> ()
        n719 = local write "milliseconds to wait"(w753) -> ()
        n720 = local write "dt"(w752) -> ()
        n721 = local write "kp"(w751) -> ()
        n722 = local write "ki"(w750) -> ()
        n723 = local write "kd"(w749) -> ()
        n724 = local write "max_step_change"(w748) -> ()
        n725 = local write "max_amplitude"(w747) -> ()
        n726 = local write "min_amplitude"(w746) -> ()
        n727 = local write "startup_cmd"(w745) -> ()
      }
    }
    n728 = local read "USER ID"() -> (w709:string)
    n729 = local write "tested by 2"(w709) -> ()
    n730 = local read "run test Calibration"() -> (w697:bool)
    n731 = local read "START TEMP"() -> (w696:bool)
    n732 = local read "Point 1 - 0.2 mm"() -> (w708:bool)
    n733 = local read "Point 2 - 0.4 mm"() -> (w707:bool)
    n734 = local read "Point 3 - 0.6 mm"() -> (w706:bool)
    n735 = local read "Point 4 - 0.8 mm"() -> (w705:bool)
    n736 = local read "Point 5 - 1.0 mm"() -> (w704:bool)
    n737 = local read "Point 6 - 1.2 mm"() -> (w703:bool)
    n738 = And(x=w696, y=w697) -> (x .and. y?=w695:bool)
    n739 = And(x=w708, y=w707) -> (x .and. y?=w702:bool)
    n740 = And(x=w706, y=w705) -> (x .and. y?=w701:bool)
    n741 = And(x=w704, y=w703) -> (x .and. y?=w699:bool)
    n742 = case shown="True" w695 {
      frame False {
        w715 = TRUE ("PAUSE")
        n743 = call "ELAPSED TIMER VI - Calibration.vi"("RESET"=w715, "PAUSE"=w715) -> ()  [unwired: 7 in, 3 out]
      }
      frame True {
        w718 = FALSE ("PAUSE")
        n744 = call "ELAPSED TIMER VI - Calibration.vi"("TARGET"=60.0, "RESET"=w718, "PAUSE"=w718) -> ("ELAPSED INDICATION"=w716:bool)  [unwired: 6 in, 2 out]
        n745 = case shown="True" w716 {
          frame False {
          }
          frame True {
            n746 = stacked-sequence {
              frame #0 {
                n747 = local write "START TEMP"(FALSE ("START TEMP")) -> ()
              }
              frame #1 {
                n748 = Wait (ms)(milliseconds to wait=u32 1500) -> ()  [unwired: 1 out]
              }
              frame #2 {
                n749 = local write "Due Write"("VC;0") -> ()
              }
              frame #3 {
                n750 = Wait (ms)(milliseconds to wait=u32 1500) -> ()  [unwired: 1 out]
              }
              frame #4 {
                n751 = local write "Due Write"("VC;0") -> ()
              }
            }
          }
        }
      }
    }
    n752 = And(x=w702, y=w701) -> (x .and. y?=w700:bool)
    n753 = And(x=w700, y=w699) -> (x .and. y?=w698:bool)
    n754 = case shown="False" w698 {
      frame False {
        n755 = property on="Accept & Save" class="Bool (strict)"("DisabledEnum"=T19."Disabled" ("Disabled")) -> ()  [unwired: 2 in, 2 out]
        n756 = property on="Tab Control 5" class="TabCtl (strict)"("Value"=enum32{"OK", "NG"}."NG" ("Tab Control 5")) -> ()  [unwired: 2 in, 2 out]
      }
      frame True {
        n757 = property on="Accept & Save" class="Bool (strict)"("DisabledEnum"=T19."Enabled" ("Disabled")) -> ()  [unwired: 2 in, 2 out]
        n758 = property on="Tab Control 5" class="TabCtl (strict)"("Value"=enum32{"OK", "NG"}."OK" ("Tab Control 5")) -> ()  [unwired: 2 in, 2 out]
      }
    }
    n759 = local read "Quit"() -> (w714:bool)
  }
  n760 = while {
    shift-right: [w782] -> _
    shift-left: "Enum - Selector" -> [w783]
    stop <- w784 stop-if-true
    # "Auto Start Logic Loop"
    n761 = case shown="\"close\"" w783 {
      tunnel: [w787 w793 w820 w852 w882 Auto_Start_enum."Exit" ("Enum - Selector") Auto_Start_enum."Init" ("Enum - Selector")] -> w782
      frame "Init", Default {
        n762 = local read "Auto Start Test"() -> (w786:bool)
        n763 = Select(t=Auto_Start_enum."Humidity & Temperature On" ("Enum - Selector"), s=w786, f=Auto_Start_enum."Init") -> (s? t:f=w787:T15)
      }
      frame "Humidity & Temperature On" {
        n764 = stacked-sequence {
          tunnel: [_ _ _ _ _ _ Auto_Start_enum."Reach point" ("Enum - Selector")] -> w790
          frame #0 {
            w795 = T19."Disabled and Grayed Out" ("Disabled")
            w796 = TRUE ("Heater Button")
            n765 = property on="Humidity" class="Bool (strict)"("DisabledEnum"=w795) -> ()  [unwired: 2 in, 2 out]
            n766 = property on="Heater Button" class="Bool (strict)"("DisabledEnum"=w795) -> ()  [unwired: 2 in, 2 out]
            n767 = local write "Heater Button"(w796) -> ()
            n768 = local write "Humidity"(w796) -> ()
            n769 = property on="Heater Button" class="Bool (strict)"("Val(Sgnl)"=TRUE ("Value (Signaling)")) -> ()  [unwired: 2 in, 2 out]
          }
          frame #1 {
            n770 = Wait (ms)(milliseconds to wait=u32 3000) -> ()  [unwired: 1 out]
          }
          frame #2 {
            n771 = local read "Set Temp"() -> (w802:dbl)
            n772 = Number To Fractional String(number=w802, precision (6)=i16 2) -> (F-format string=w799:string)  [unwired: 2 in]
            n773 = Concatenate Strings("ST;" ("Command"), w799) -> (w800:string)
            n774 = local write "Due Write"(w800) -> ()
          }
          frame #3 {
            n775 = Wait (ms)(milliseconds to wait=u32 1500) -> ()  [unwired: 1 out]
          }
          frame #4 {
            (unwired) i16 2 ("precision (6)")
            n776 = local read "WriteHumidity"() -> (w804:string[])
            n777 = local read "Set Rh"() -> (w807:dbl)
            n778 = Number To Fractional String(number=w807) -> (F-format string=w808:string)  [unwired: 3 in]
            n779 = Concatenate Strings("M;" ("new element/subarray"), w808) -> (w809:string)
            n780 = Insert Into Array(array=w804, new element=w809) -> (w805:string[])  [unwired: 1 in]
            n781 = local write "WriteHumidity"(w805) -> ()
            n782 = local write "Due Write"("HE;1" ("Command")) -> ()
          }
          frame #5 {
            n783 = Wait (ms)(milliseconds to wait=u32 1500) -> ()  [unwired: 1 out]
          }
          frame #6 {
            w812 = TRUE ("Reach point temp")
            n784 = local write "Reach point Humidity"(w812) -> ()
            n785 = local write "Reach point temp"(w812) -> ()
          }
        }
        n786 = local read "Auto Start Test"() -> (w792:bool)
        n787 = Not(x=w792) -> (.not. x?=w791:bool)
        n788 = Select(t=Auto_Start_enum."close", s=w791, f=w790) -> (s? t:f=w793:T15)
      }
      frame "Reach point" {
        w821 = TRUE ("PAUSE")
        w829 = 1.0 ("y")
        w832 = 1.0 ("y")
        n789 = local read "Set Temp"() -> (w814:dbl)
        n790 = local read "Set Humidity:"() -> (w828:dbl)
        n791 = local read "Humidity ( %RH )"() -> (w833:dbl)
        n792 = Add(x=w814, y=w832) -> (x+y=w831:dbl)
        n793 = Subtract(x=w814, y=w832) -> (x-y=w830:dbl)
        n794 = Add(x=w828, y=w829) -> (x+y=w827:dbl)
        n795 = Subtract(x=w828, y=w829) -> (x-y=w826:dbl)
        n796 = local read "TEMP"() -> (w834:dbl)
        n797 = In Range and Coerce(upper limit=w827, x=w833, lower limit=w826) -> (In Range?=w815:bool)  [unwired: 1 out]
        n798 = In Range and Coerce(upper limit=w831, x=w834, lower limit=w830) -> (In Range?=w816:bool)  [unwired: 1 out]
        n799 = case shown="True" w815 {
          frame False {
          }
          frame True {
            n800 = case shown="True" "Reach point Humidity" {
              selector: "Reach point Humidity" -> [_ w840]
              frame False {
              }
              frame True {
                n801 = local read "EVENT LOG"() -> (w837:string)
                n802 = Not(x=w840) -> (.not. x?=w839:bool)
                n803 = local write "Reach point Humidity"(w839) -> ()
                n804 = call "Event Log.vi"("Content"="Target Humidity reached", "EVENT LOG"=w837) -> ("EVENT LOG"=w838:string)  [unwired: 8 in, 1 out]